vi "IMAQdx_AbsImage_Flea3_v4.3.vi"() -> ()   [LabVIEW 2012]
doc: "Take a single PixelFly exposure and display the result as an intensity graph.This VI illustrates the basics of taking an exposure with the PixelFly camera. Use Ctrl-H to get help on any of the controls\n\nCopyright 2001, The Cooke Corporation."
uses:
  LabVIEW Data V4.10/Shared Libraries/Controls/FileName_Cluster.ctl
  <vilib>/userdefined/High Color/IMAQdx.ctl
  <vilib>/vision/driver/IMAQdx.llb/IMAQdx Acquisition Mode.ctl
  Shared Libraries/Controls/FileInfo_Global.vi
  <vilib>/Analysis/NI_AALBase.lvlib
  <vilib>/vision/driver/NI_Vision_Acquisition_Software.lvlib
panel:
  in  "Interrupt":bool
  out "Buffer Number":u32=4294967294
  out "Frames":i32
  out "Loop":i32=292
  out "Status":string="Running..."
  in  "stop":bool
  in  "Tab Control":enum32{"Setup", "Images", "Hardware status"}(tab)=enum."Images"
  in  "Camera Name":T1="Flr XZ"
  in  "Experiment":T2(ring)=enum."Sr"
  in  "Accept parameters from remote system":bool=TRUE
  in  "Bias (Amps)":dbl
  in  "Pinch Coil (Amps)":dbl=520.0
  in  "Expansion time (ms)":dbl=19.0
  in  "Trap min at 0 (MHz)":dbl=2.85
  in  "Detuning (Linewidths)":dbl
  in  "Racetrack (Amps)":dbl=540.0
  in  "Magnification":dbl=0.399
  in  "Image direction":enum16{"XY", "XZ"}(ring)=enum."XZ"
  in  "Imaging technique":enum16{"Absorption", "Fluorescence", "RawImage"}(ring)
  in  "File Parameters":T3={"Data Root"=path "C:/Experiment/Data", "Index"=20503, "Instrument"="Flea3_20S4M"} {"Index" format="%04d"}
  in  "Send data to Igor?":bool=TRUE
  out "Command to Igor":string="AutoRunV3(\"rMOTDet_Sr_88\",\"C:\\\\Experiment\\\\Data\\\\2013\\\\October\\\\09\\\\Flea3_20S4M_09Oct2013_20502.ibw\") "
  out "Image note":string="Experiment=Sr\nCamera_ID=Flea3_20S4M\nImageType=Raw\nDataType=Absorption\nImageDirection=XZ\nMagnification=3.990000E-1\nFileNumber=20502\n# Current Variables\n# \nplus_zman=-1.971000E+0\nminus_zman=-1.584000E+0\ncompensation=-8.000000E-1\nXshim=4.000000E-1\nYshim=1.200000E+0\nZshim=9.000000E-1\nProbePow=1.600000E+0\ntau=0.000000E+0\ntEnd=0.000000E+0\nDipStart=0.000000E+0\nMOTcurrent=-1.500000E+0\nProbeDet=0.000000E+0\nTOF=1.000000E-4\nMOTPow=8.000000E+0\nMOTdetuning=-4.500000E+1\nRampTau=2.000000E-3\nPf=1.900000E+0\nrMOTcurr=-7.500000E-2\nrMOTcurrI=-5.000000E-2\nrMOTcurrF=-5.000000E-2\ncombWidthI=4.000000E+0\ncombWidthF=5.000000E-1\nrMOTbroadDetuning=2.750000E+0\nrMOTsat1=1.500000E+4\nrMOTsat2=1.000000E+3\nrMOTsat3=1.500000E+2\nsingleFreqDet=1.000000E+3\nPdet=3.500000E+0\nZshimVar=9.000000E-1\n# Master Staging List\n# Line\tMarker\tOption\tHalt\t0       4       8      12      16      20    AO\tDelay\t\tPoints\t0\t\t1\t\t2\t\t3\t\t4\t\t5\t\t6\t\t7\t\t8\t\t9\t\t10\t\t11\t\t12\t\t13\t\t14\t\t15\t\tComment\n00\t\tRamp\t1 0 0 0 0 0 1 0 0 0 1 1 1 1 1 0 0 0 0 0 0 0 0 0\t.1\t0\tplus_zman\tminus_zman\tcompensation\tMOTcurrent\trMOTsat(rMOTsat1)\tcombAmplitude(combWidthI)\trMOTdelta(-(rMOTbroadDetuning +combWidthI/2))\t2.65\tbMOTdelta(MOTdetuning)\tbMOTpow(0.5)\tProbePow\tPdelta(Pdet)\tXshim\tYshim\tZshim\t0\treset\n01\t\tRamp\t1 1 0 0 0 0 0 0 0 0 1 1 1 1 1 1 0 0 0 0 0 0 0 0\t3\t0\tplus_zman\tminus_zman\tcompensation\tMOTcurrent\trMOTsat(rMOTsat1)\tcombAmplitude(combWidthI)\trMOTdelta(-(rMOTbroadDetuning +combWidthI/2))\t2.65\tbMOTdelta(MOTdetuning)\tbMOTpow(MOTPow)\tProbePow\tPdelta(Pdet)\tXshim\tYshim\tZshim\t0\tblue MOT load\n02\t\tRamp\t1 1 0 0 0 0 0 0 0 0 1 1 1 1 1 1 0 0 0 0 0 0 0 0\t0.000244\t0\tplus_zman\tminus_zman\tcompensation\tMOTcurrent\trMOTsat(rMOTsat1)\tcombAmplitude(combWidthI)\trMOTdelta(-(rMOTbroadDetuning +combWidthI/2))\t2.65\tbMOTdelta(MOTdetuning)\tbMOTpow(MOTPow)\tProbePow\tPdelta(Pdet)\tXshim\tYshim\tZshim\t0\tpretrig\n03\t\tRamp\t1 1 0 0 0 0 0 0 0 0 1 1 1 1 1 1 0 0 0 0 0 0 0 0\t0.074\t0\tplus_zman\tminus_zman\tcompensation\tMOTcurrent\trMOTsat(rMOTsat1)\tcombAmplitude(combWidthI)\trMOTdelta(-(rMOTbroadDetuning +combWidthI/2))\t2.65\tbMOTdelta(MOTdetuning)\tbMOTpow(MOTPow)\tProbePow\tPdelta(Pdet)\tXshim\tYshim\tZshim\t0\tCamWaitTime\n04\t\tRamp\t1 1 0 0 0 0 0 0 0 0 1 1 1 1 1 1 0 0 0 0 0 0 0 0\t0.001120\t0\tplus_zman\tminus_zman\tcompensation\tMOTcurrent\trMOTsat(rMOTsat1)\tcombAmplitude(combWidthI)\trMOTdelta(-(rMOTbroadDetuning +combWidthI/2))\t2.65\tbMOTdelta(MOTdetuning)\tbMOTpow(MOTPow)\tProbePow\tPdelta(Pdet)\tXshim\tYshim\tZshim\t0\tProbeShutOn\n05\t\tRamp\t1 1 0 0 0 0 0 0 0 0 1 1 1 1 1 1 0 0 0 0 0 0 0 0\t0.000260\t0\tplus_zman\tminus_zman\tcompensation\tMOTcurrent\trMOTsat(rMOTsat1)\tcombAmplitude(combWidthI)\trMOTdelta(-(rMOTbroadDetuning +combWidthI/2))\t2.65\tbMOTdelta(MOTdetuning)\tbMOTpow(MOTPow)\tProbePow\tPdelta(Pdet)\tXshim\tYshim\tZshim\t0\tRepumpShutOff\n06\t\tRamp\t1 1 0 0 0 0 1 0 0 0 1 1 1 1 1 1 0 0 0 0 0 0 0 0\t0.001370\t0\tplus_zman\tminus_zman\tcompensation\tMOTcurrent\trMOTsat(rMOTsat1)\tcombAmplitude(combWidthI)\trMOTdelta(-(rMOTbroadDetuning +combWidthI/2))\t2.65\tbMOTdelta(MOTdetuning)\tbMOTpow(MOTPow)\tProbePow\tPdelta(Pdet)\tXshim\tYshim\tZshim\t0\tMOTShutOff\n07\t\tRamp\t1 1 0 0 0 0 1 0 0 0 1 1 1 1 0 0 0 0 0 0 0 0 0 0\t0.000230\t0\tplus_zman\tminus_zman\tcompensation\trMOTcurrI\trMOTsat(rMOTsat1)\tcombAmplitude(combWidthI)\trMOTdelta(-(rMOTbroadDetuning +combWidthI/2))\t2.65\tbMOTdelta(MOTdetuning)\tbMOTpow(0.5)\tProbePow\tPdelta(Pdet)\tXshim\tYshim\tZshim\t0\tCoil Switch\n08\t\tRamp\t1 1 0 0 0 0 1 0 0 0 1 1 0 0 0 0 0 0 0 0 0 0 0 0\t.1\t0\tplus_zman\tminus_zman\tcompensation\trMOTcurrI\trMOTsat(rMOTsat1)\tcombAmplitude(combWidthI)\trMOTdelta(-(rMOTbroadDetuning +combWidthI/2))\t2.65\tbMOTdelta(MOTdetuning)\tbMOTpow(0.5)\tProbePow\tPdelta(Pdet)\tXshim\tYshim\tZshim\t0\tCapture Red MOT\n09\t\tRamp\t1 1 0 0 0 0 1 0 0 0 1 1 0 0 0 0 0 0 0 0 0 0 0 0\t.1\t0\tplus_zman\tminus_zman\tcompensation\trMOTcurrI\tLineRamp(f,rMOTsat(rMOTsat1),rMOTsat(rMOTsat2))\tLineRamp(f,combAmplitude(combWidthI),combAmplitude(combWidthF))\tLineRamp(f,rMOTdelta(-(rMOTbroadDetuning +combWidthI/2)),rMOTdelta(-(rMOTbroadDetuning +combWidthF/2)))\t2.65\tbMOTdelta(MOTdetuning)\tbMOTpow(0.5)\tProbePow\tPdelta(Pdet)\tXshim\tYshim\tZshim\t0\tRamp broad rMOT\n10\t\tRamp\t1 1 0 0 0 0 1 0 0 0 1 1 0 0 0 0 0 0 0 0 0 0 0 0\t.05\t0\tplus_zman\tminus_zman\tcompensation\trMOTcurrI\trMOTsat(rMOTsat2)\tcombAmplitude(combWidthF)\trMOTdelta(-(rMOTbroadDetuning +combWidthF/2))\t2.65\tbMOTdelta(MOTdetuning)\tbMOTpow(0.5)\tProbePow\tPdelta(Pdet)\tXshim\tYshim\tLineRamp(f,Zshim,ZshimVar)\t0\tRamp broad rMOT\n11\t\tRamp\t1 1 0 0 0 0 1 0 0 0 1 1 0 0 0 0 0 0 0 0 0 0 0 0\t.1\t0\tplus_zman\tminus_zman\tcompensation\trMOTcurrI\trMOTsat(rMOTsat2)\tcombAmplitude(combWidthF)\trMOTdelta(-(rMOTbroadDetuning +combWidthF/2))\t2.65\tbMOTdelta(MOTdetuning)\tbMOTpow(0.5)\tProbePow\tPdelta(Pdet)\tXshim\tYshim\tZshimVar\t0\tRamp broad rMOT\n12\t\tRamp\t1 1 0 0 0 0 1 1 1 1 0 1 0 0 0 0 0 0 0 0 0 0 0 0\tTOF\t0\tplus_zman\tminus_zman\tcompensation\trMOTcurrF\trMOTsat(rMOTsat3)\tcombAmplitude(combWidthF)\trMOTdelta(-(rMOTbroadDetuning +combWidthF/2))\t2.65\tbMOTdelta(MOTdetuning)\tbMOTpow(0.5)\tProbePow\tPdelta(Pdet)\tXshim\tYshim\tZshimVar\t0\tTOF\n13\t\tRamp\t1 1 0 0 0 0 1 1 1 1 0 1 0 0 0 0 0 0 0 0 0 0 0 0\t.000044\t0\tplus_zman\tminus_zman\tcompensation\trMOTcurrF\trMOTsat(rMOTsat3)\tcombAmplitude(combWidthI)\trMOTdelta(-(rMOTbroadDetuning +combWidthI/2))\t2.65\tbMOTdelta(MOTdetuning)\tbMOTpow(0.5)\tProbePow\tPdelta(Pdet)\tXshim\tYshim\tZshimVar\t0\tarm camera\n14\t\tRamp\t1 1 0 0 0 0 1 1 1 1 0 1 0 1 0 0 0 0 0 0 0 0 0 0\t.000200\t0\tplus_zman\tminus_zman\tcompensation\trMOTcurrF\trMOTsat(rMOTsat3)\tcombAmplitude(combWidthI)\trMOTdelta(-(rMOTbroadDetuning +combWidthI/2))\t2.65\tbMOTdelta(MOTdetuning)\tbMOTpow(0.5)\tProbePow\tPdelta(Pdet)\tXshim\tYshim\tZshimVar\t0\tatom img\n15\t\tRamp\t1 0 0 0 0 0 1 1 1 1 1 1 0 0 0 0 0 0 0 0 0 0 0 0\t.07\t0\tplus_zman\tminus_zman\tcompensation\trMOTcurrF\trMOTsat(rMOTsat3)\tcombAmplitude(combWidthI)\trMOTdelta(-(rMOTbroadDetuning +combWidthI/2))\t2.65\tbMOTdelta(MOTdetuning)\tbMOTpow(0.5)\tProbePow\tPdelta(Pdet)\tXshim\tYshim\tZshimVar\t0\ttransmit img\n16\t\tRamp\t0 0 0 0 0 0 1 1 1 1 1 1 0 0 1 1 0 0 0 0 0 0 0 0\t.000044\t0\tplus_zman\tminus_zman\tcompensation\trMOTcurrF\trMOTsat(rMOTsat3)\tcombAmplitude(combWidthI)\trMOTdelta(-(rMOTbroadDetuning +combWidthI/2))\t2.65\tbMOTdelta(MOTdetuning)\tbMOTpow(0.5)\tProbePow\tPdelta(Pdet)\tXshim\tYshim\tZshimVar\t0\tarm camera\n17\t\tRamp\t0 0 0 0 0 0 1 1 1 1 1 1 0 1 1 1 0 0 0 0 0 0 0 0\t.000200\t0\tplus_zman\tminus_zman\tcompensation\trMOTcurrF\trMOTsat(rMOTsat1)\tcombAmplitude(combWidthI)\trMOTdelta(-(rMOTbroadDetuning +combWidthI/2))\t2.65\tbMOTdelta(MOTdetuning)\tbMOTpow(0.5)\tProbePow\tPdelta(Pdet)\tXshim\tYshim\tZshimVar\t0\tprobe img\n18\t\tRamp\t0 0 0 0 0 0 1 1 1 1 1 1 0 0 1 1 0 0 0 0 0 0 0 0\t.07\t0\tplus_zman\tminus_zman\tcompensation\trMOTcurrF\trMOTsat(rMOTsat1)\tcombAmplitude(combWidthI)\trMOTdelta(-(rMOTbroadDetuning +combWidthI/2))\t2.65\tbMOTdelta(MOTdetuning)\tbMOTpow(0.5)\tProbePow\tPdelta(Pdet)\tXshim\tYshim\tZshimVar\t0\ttransmit img\n19\t\tRamp\t0 0 0 0 0 0 1 1 1 1 1 1 0 0 1 1 0 0 0 0 0 0 0 0\t.000044\t0\tplus_zman\tminus_zman\tcompensation\trMOTcurrF\trMOTsat(rMOTsat1)\tcombAmplitude(combWidthI)\trMOTdelta(-(rMOTbroadDetuning +combWidthI/2))\t2.65\tbMOTdelta(MOTdetuning)\tbMOTpow(0.5)\tProbePow\tPdelta(Pdet)\tXshim\tYshim\tZshimVar\t0\tarm camera\n20\t\tRamp\t0 0 0 0 0 0 1 1 1 1 1 1 0 0 1 1 0 0 0 0 0 0 0 0\t.000200\t0\tplus_zman\tminus_zman\tcompensation\trMOTcurrF\trMOTsat(rMOTsat1)\tcombAmplitude(combWidthI)\trMOTdelta(-(rMOTbroadDetuning +combWidthI/2))\t2.65\tbMOTdelta(MOTdetuning)\tbMOTpow(0.5)\tProbePow\tPdelta(Pdet)\tXshim\tYshim\tZshimVar\t0\tbg img\n21\t\tRamp\t0 0 0 0 0 0 1 1 1 1 1 1 0 0 1 1 0 0 0 0 0 0 0 0\t.07\t0\tplus_zman\tminus_zman\tcompensation\tMOTcurrent\trMOTsat(rMOTsat1)\tcombAmplitude(combWidthI)\trMOTdelta(-(rMOTbroadDetuning +combWidthI/2))\t2.65\tbMOTdelta(MOTdetuning)\tbMOTpow(0.5)\tProbePow\tPdelta(Pdet)\tXshim\tYshim\tZshimVar\t0\ttransmit img\n22\t\tRamp\t0 0 0 0 0 0 1 0 0 0 1 1 1 1 1 1 0 0 0 0 0 0 0 0\t0.5\t0\tplus_zman\tminus_zman\tcompensation\tMOTcurrent\trMOTsat(rMOTsat1)\tcombAmplitude(combWidthI)\trMOTdelta(-(rMOTbroadDetuning +combWidthI/2))\t2.65\tbMOTdelta(MOTdetuning)\tbMOTpow(MOTPow)\tProbePow\tPdelta(Pdet)\tXshim\tYshim\tZshimVar\t0\talignment\n# Slave Staging List\n# Line\tMarker\tOption\tHalt\t0       4       8      12      16      20    AO\tDelay\t\tPoints\t0\t\t1\t\t2\t\t3\t\t4\t\t5\t\t6\t\t7\t\t8\t\t9\t\t10\t\t11\t\t12\t\t13\t\t14\t\t15\t\tComment\n# SRS List\n# \n#\n# Evaporation\n\nDDS Table\r\n"
  in  "Igor Wave Name":string="Test_Img"
  in  "Save file to archive?":bool=TRUE
  in  "Timeout (ms)":u32=10000
  in  "Gain":dbl
  in  "Shutter speed":dbl=0.03
  out "Timeout":bool=TRUE
  out "Trigger Overrun":bool=TRUE
  in  "Quad [Amps]":dbl=540.0
  in  "Source of File Data":refnum<k21>="\\\\Control\\VariableLibrary\\Instruction String"
  in  "Bits to shift":i32
  in  "Raw image to view":u16(ring)=1 items=["Clear", "Absorbtion", "Probe", "Background"]
  in  "Update Graphics":bool=TRUE
  out "Raw Image":u16[][](graph)
  out "Processed Image":sgl[][](graph)
  out "Histogram":cluster{"X Values":dbl[], dbl[]}(graph)={"X Values"=[33.3203125, 83.9609375, 134.6015625, 185.2421875, 235.8828125, 286.5234375, 337.1640625, 387.8046875, 438.4453125, 489.0859375, 539.7265625, 590.3671875, 641.0078125, 691.6484375, 742.2890625, 792.9296875, 843.5703125, 894.2109375, 944.8515625, 995.4921875, 1046.1328125, 1096.7734375, 1147.4140625, 1198.0546875, 1248.6953125, 1299.3359375, 1349.9765625, 1400.6171875, 1451.2578125, 1501.8984375, 1552.5390625, 1603.1796875, 1653.8203125, 1704.4609375, 1755.1015625, 1805.7421875, 1856.3828125, 1907.0234375, 1957.6640625, 2008.3046875, 2058.9453125, 2109.5859375, 2160.2265625, 2210.8671875, 2261.5078125, 2312.1484375, 2362.7890625, 2413.4296875, 2464.0703125, 2514.7109375, 2565.3515625, 2615.9921875, 2666.6328125, 2717.2734375, 2767.9140625, 2818.5546875, 2869.1953125, 2919.8359375, 2970.4765625, 3021.1171875, 3071.7578125, 3122.3984375, 3173.0390625, 3223.6796875], [3.7989267385772014, 4.5429374082326195, 4.748110467494984, 4.839886381275089, 4.874528201815916, 4.882473307537075, 4.900061102735481, 4.901899475590769, 4.901322072145771, 4.91365493508662, 4.918664530902084, 4.913633741719355, 4.9192611900011745, 4.903768042526874, 4.9022368466531665, 4.881578647766411, 4.85617283090403, 4.839697967180202, 4.816519689651045, 4.788479480483438, 4.776606761880874, 4.7497285878404885, 4.705264862317404, 4.681819910988056, 4.644999560017717, 4.606370615114146, 4.576064788225377, 4.5289423974157295, 4.494182432516058, 4.452629651622018, 4.390139938467622, 4.355432362470549, 4.299746933493803, 4.233478391931892, 4.179666668690498, 4.114377429786155, 4.018325945402921, 3.9655309436228605, 3.874423830586502, 3.8100307864058394, 3.713994267660644, 3.6097011023793995, 3.5090680450171616, 3.3694014136966244, 3.248218561190075, 3.118264726089479, 2.9836262871245345, 2.8228216453031045, 2.6748611407378116, 2.53655844257153, 2.342422680822206, 2.173186268412274, 2.0253058652647704, 1.7993405494535817, 1.5797835966168101, 1.146128035678238, 1.2304489213782739, 0.6020599913279624, 0.8450980400142568, 0.8450980400142568, 0.9030899869919435, 0.8450980400142568, 0.0, 0.47712125471966244]}
  out "Images":u16[][][](array[numeric])
  out "Camera Error":errorcluster={"status"=FALSE, "code"=-1074360293, "source"="IMAQdx Get Image.vi"}
  out "DDE Error":errorcluster={"status"=FALSE, "code"=0, "source"="DDE Close: No Error"}
  out "Status Array":T4(array[cluster])=[{"AcquisitionInProgress"=FALSE, "BufferCount"=4, "LastBufferNumber"=3, "LostBufferCount"=0}, {"AcquisitionInProgress"=TRUE, "BufferCount"=1, "LastBufferNumber"=0, "LostBufferCount"=0}, {"AcquisitionInProgress"=TRUE, "BufferCount"=2, "LastBufferNumber"=1, "LostBufferCount"=0}, {"AcquisitionInProgress"=TRUE, "BufferCount"=3, "LastBufferNumber"=2, "LostBufferCount"=0}, {"AcquisitionInProgress"=TRUE, "BufferCount"=4, "LastBufferNumber"=3, "LostBufferCount"=0}]
  # "Flea3 Image Acquisition v4.3"
  # "Experimental Paramaters"
  # "Cam0 is XZ, Cam1 is XY"
  # "RbYb: set to 0."
  # "The only get set on 1st run.\nUse  a Gain of 10:\n* Seems to give a readout error of 1 bit.\n* Know intensity calibration"
  # "In both techniques 3 images\nare aquired, but in Fluorescense\nthe 3rd is discarded"
  # "Sr: .663  is XZ\n     5.48 is XY"
  # "Obsolete: (now done with network variables)\nWhen paramaters are accepted from a remote system a DataSockets server\nmust be running on this machine (in start menu in National Instruments folder)"
  # "Camera configuration"
  # "File configuration"
  # "When the gain is 10 :  742 counts = Isat with 100 us pulse.  This is fine and\nis the point of highest SNR.  Linearized in software."
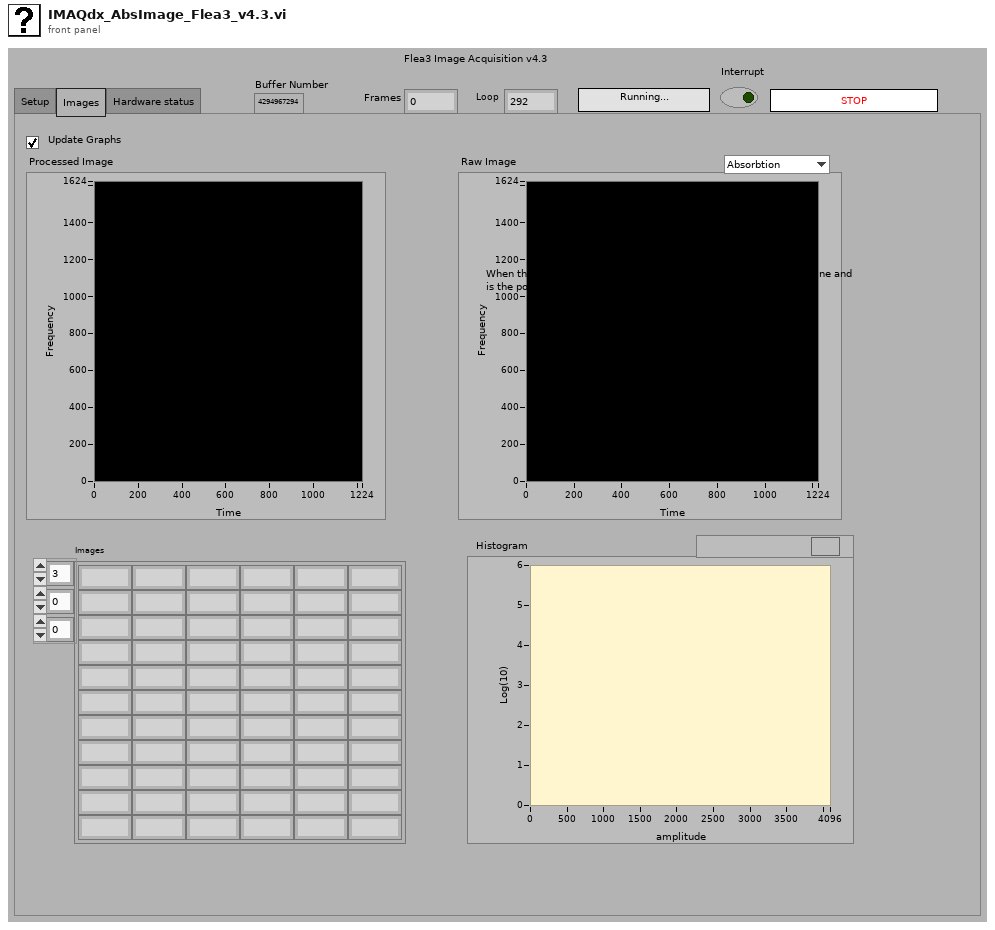
[diagram p1: front panel]
types:
  T1 = typedef "IMAQdx.ctl" = refnum<k21>
  T2 = enum16{"Rubidium I", "Rubidium II", "RbLi", "RbYb", "Sr"}
  T3 = typedef "FileName_Cluster.ctl" = cluster{"Data Root":path, "Index":u32, "Instrument":string}
  T4 = cluster{"AcquisitionInProgress":bool, "BufferCount":u32, "LastBufferNumber":u32, "LostBufferCount":u32}[]
  T5 = typedef "NI_Vision_Acquisition_Software.lvlib/IMAQdx Acquisition Mode.ctl" = enum32{"One Shot", "Continuous"}
  T6 = typedef "Image Type" = u32
  T7 = typedef "IMAQ Image.ctl" = refnum<image>
  T8 = cluster{"AcquisitionInProgress":bool, "BufferCount":u32, "LastBufferNumber":u32, "LostBufferCount":u32}
  T9 = cluster{"X Values":dbl[], "Histogram: h(x)":i32[]}
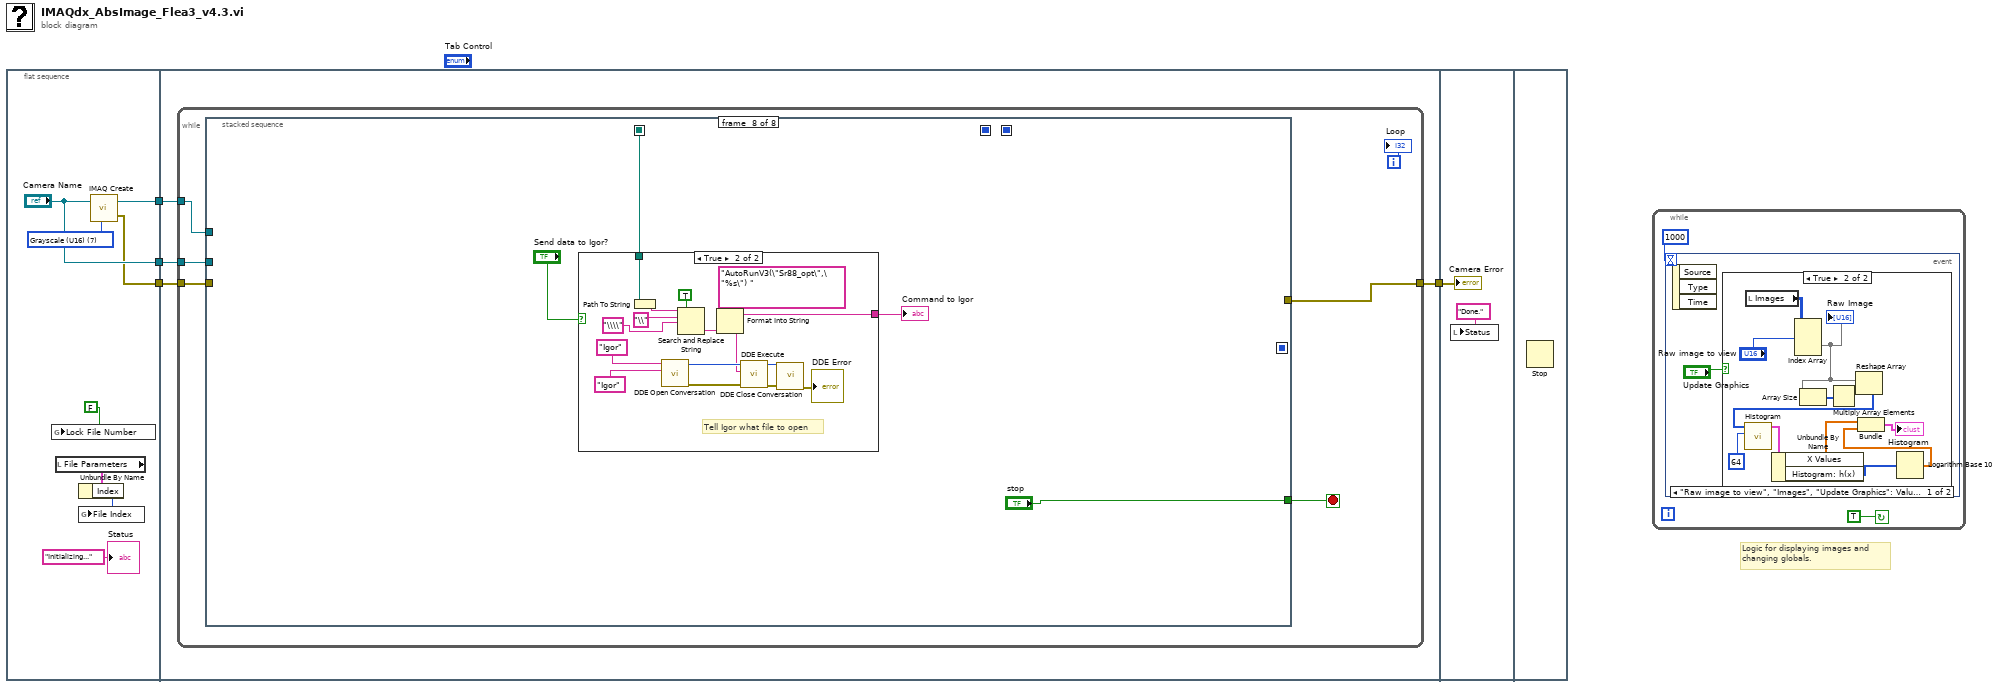
[diagram p0: block diagram]
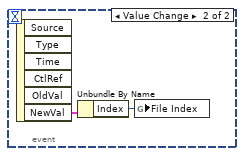
[diagram p3: hidden frame]
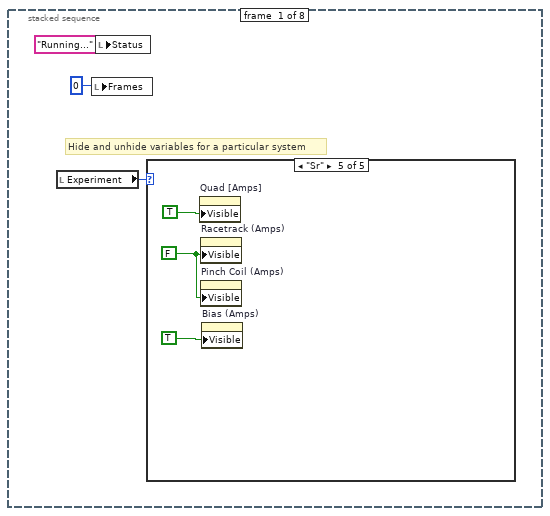
[diagram p4: hidden frame]
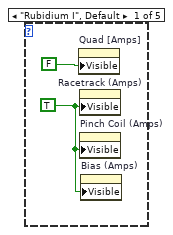
[diagram p5: hidden frame]
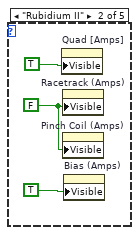
[diagram p6: hidden frame]
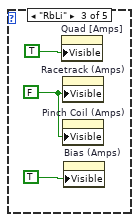
[diagram p7: hidden frame]
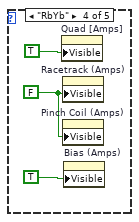
[diagram p8: hidden frame]
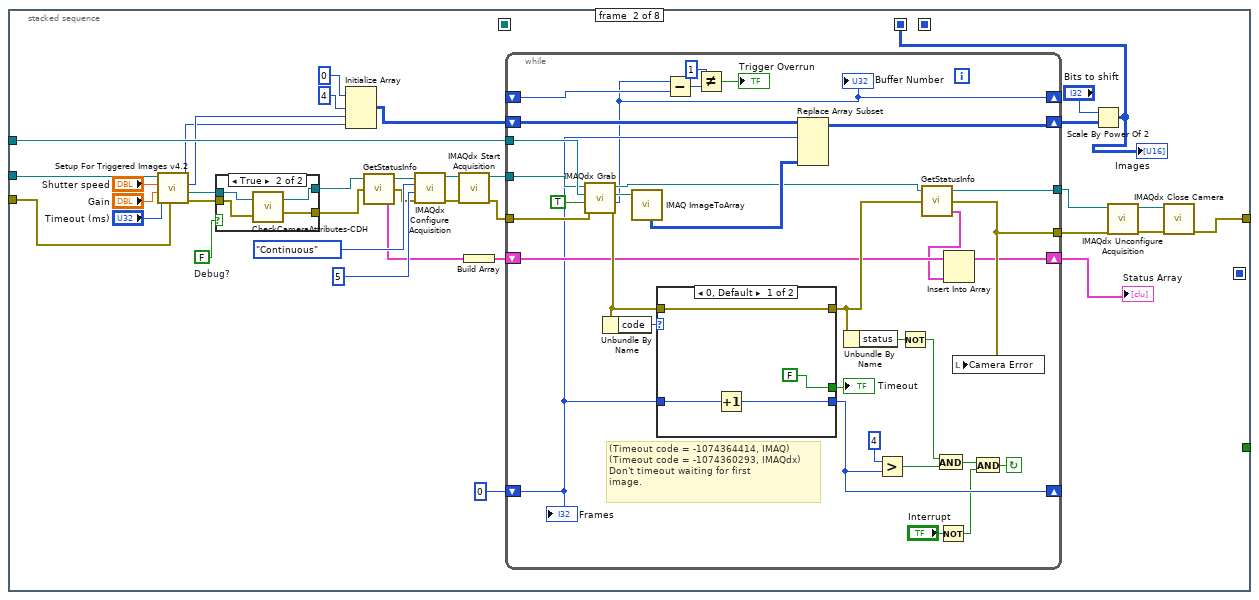
[diagram p9: hidden frame]
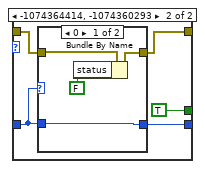
[diagram p11: hidden frame]
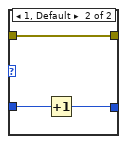
[diagram p12: hidden frame]
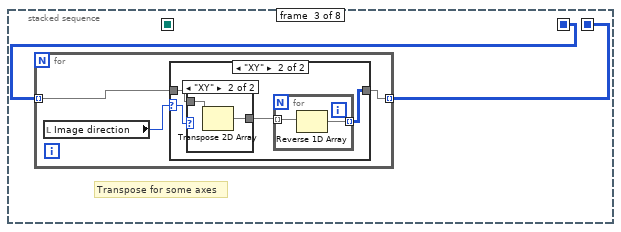
[diagram p13: hidden frame]
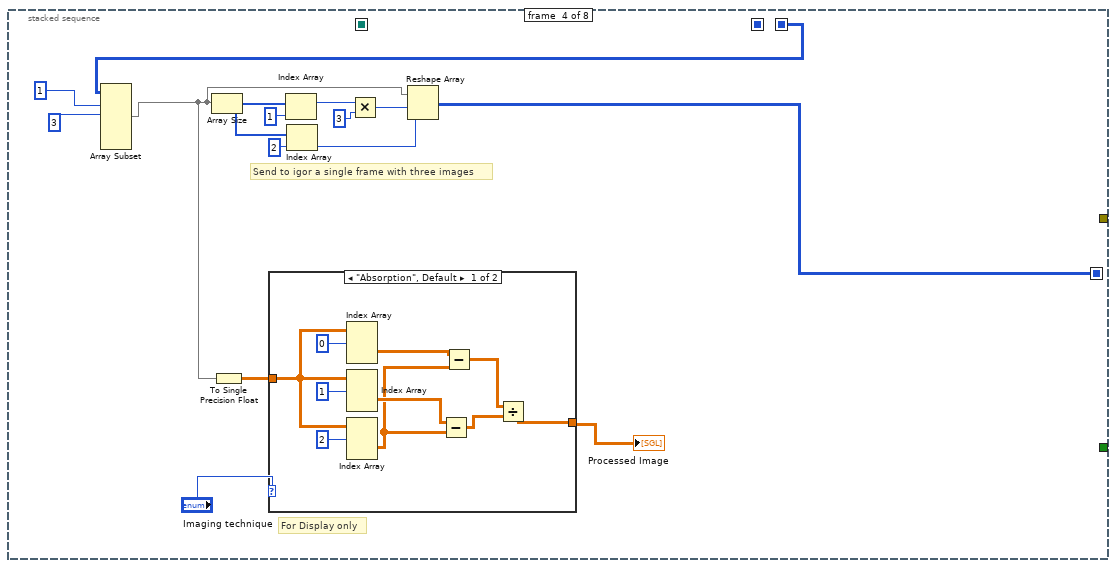
[diagram p16: hidden frame]
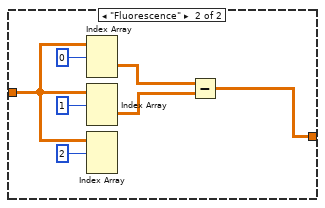
[diagram p17: hidden frame]
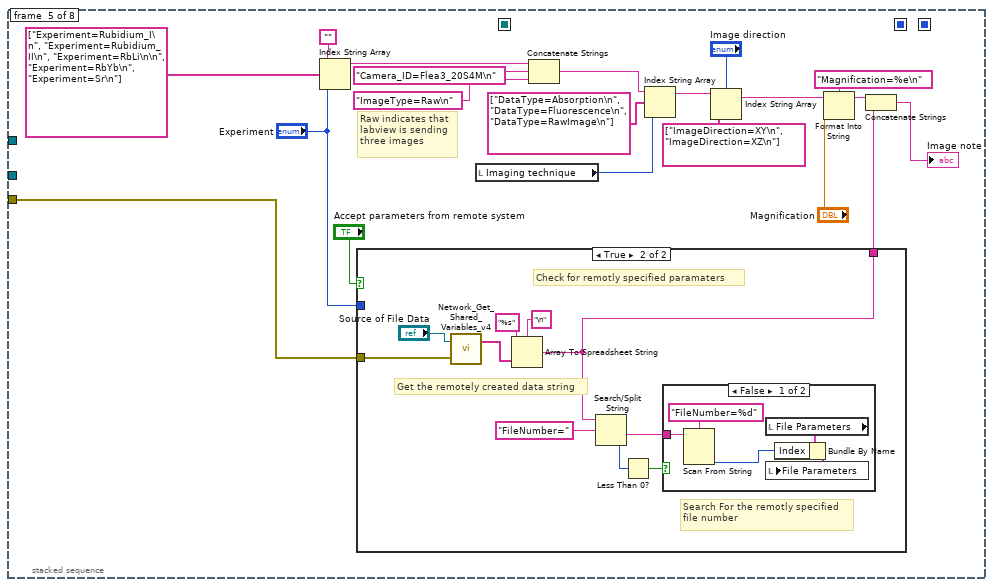
[diagram p18: hidden frame]
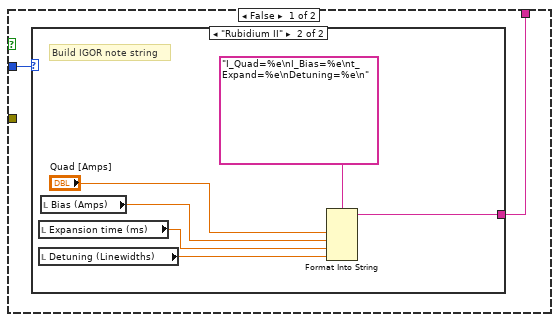
[diagram p19: hidden frame]
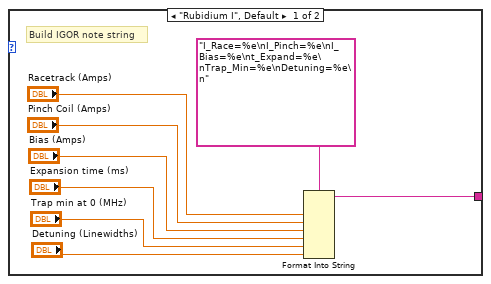
[diagram p20: hidden frame]
diagram:
  # "Logic for displaying images and\nchanging globals."
  n1 = flat-sequence {
    tunnel: [w8] -> w4
    tunnel: ["Camera Name"] -> w3
    tunnel: [w6] -> w2
    tunnel: w3 -> [w16]
    tunnel: w4 -> [w15]
    tunnel: w2 -> [w14]
    tunnel: [w13] -> w1
    tunnel: w1 -> [w261]
    frame #0 {
      w5 = T6 7 items=["Grayscale (U8)", "Grayscale (I16)", "Grayscale (SGL)", "Complex (CSG)", "RGB (U32)", "HSL (U32)", "RGB (U64)", "Grayscale (U16)"] ("Image Type")
      n2 = global write "FileInfo_Global.vi" "Lock File Number"(FALSE) -> ()
      n3 = local read "File Parameters"() -> (w9:T3)
      n4 = Unbundle By Name(w9) -> ("Index"=w10:u32)
      n5 = global write "FileInfo_Global.vi" "File Index"(w10) -> ()
      n6 = call "IMAQ Create"("Image Name"="Camera Name", "Image Type"=w5) -> ("New Image"=w8:T7, "error out"=w6:errorcluster)  [unwired: 2 in, 1 out]
      "Status" <- "Initializing..."
    }
    frame #1 {
      n7 = while {
        tunnel: w16 -> [w19]
        tunnel: w15 -> [w20]
        tunnel: w14 -> [w18]
        tunnel: [w17] -> w13
        i -> [w22]
        stop <- w21 stop-if-true
        n8 = stacked-sequence {
          seq-local: [_ _ _ w158 _ _ _ _] -> [_ _ _ _ _ w233 _ _]
          seq-local: [_ _ _ _ _ w229 _ _] -> [_ _ _ _ _ _ _ w243]
          seq-local: [_ w60 _ _ _ _ _ _] -> [_ _ w132 _ _ _ _ _]
          seq-local: [_ _ w131 _ _ _ _ _] -> [_ _ _ w149 _ _ _ _]
          tunnel: [_ _ _ _ _ _ _ "stop"] -> w21
          tunnel: w18 -> [_ w66 _ _ w185 _ _ _]
          tunnel: w19 -> [_ w67 _ _ _ _ _ _]
          tunnel: w20 -> [_ w75 _ _ _ _ _ _]
          tunnel: [_ w65 _ _ _ _ _ _] -> w17
          frame #0 {
            # "Hide and unhide variables for a particular system"
            n9 = local read "Experiment"() -> (w23:T2)
            n10 = local write "Frames"(0) -> ()
            n11 = local write "Status"("Running...") -> ()
            n12 = case shown="\"Sr\"" w23 {
              frame "Rubidium I", Default {
                w26 = TRUE
                n13 = property on="Quad [Amps]" class="DigNum (strict)"("Visible"=FALSE) -> ()  [unwired: 2 in, 2 out]
                n14 = property on="Racetrack (Amps)" class="DigNum (strict)"("Visible"=w26) -> ()  [unwired: 2 in, 2 out]
                n15 = property on="Pinch Coil (Amps)" class="DigNum (strict)"("Visible"=w26) -> ()  [unwired: 2 in, 2 out]
                n16 = property on="Bias (Amps)" class="DigNum (strict)"("Visible"=w26) -> ()  [unwired: 2 in, 2 out]
              }
              frame "Rubidium II" {
                w29 = FALSE
                n17 = property on="Quad [Amps]" class="DigNum (strict)"("Visible"=TRUE) -> ()  [unwired: 2 in, 2 out]
                n18 = property on="Racetrack (Amps)" class="DigNum (strict)"("Visible"=w29) -> ()  [unwired: 2 in, 2 out]
                n19 = property on="Pinch Coil (Amps)" class="DigNum (strict)"("Visible"=w29) -> ()  [unwired: 2 in, 2 out]
                n20 = property on="Bias (Amps)" class="DigNum (strict)"("Visible"=TRUE) -> ()  [unwired: 2 in, 2 out]
              }
              frame "RbLi" {
                w32 = FALSE
                n21 = property on="Quad [Amps]" class="DigNum (strict)"("Visible"=TRUE) -> ()  [unwired: 2 in, 2 out]
                n22 = property on="Racetrack (Amps)" class="DigNum (strict)"("Visible"=w32) -> ()  [unwired: 2 in, 2 out]
                n23 = property on="Pinch Coil (Amps)" class="DigNum (strict)"("Visible"=w32) -> ()  [unwired: 2 in, 2 out]
                n24 = property on="Bias (Amps)" class="DigNum (strict)"("Visible"=TRUE) -> ()  [unwired: 2 in, 2 out]
              }
              frame "RbYb" {
                w35 = FALSE
                n25 = property on="Quad [Amps]" class="DigNum (strict)"("Visible"=TRUE) -> ()  [unwired: 2 in, 2 out]
                n26 = property on="Racetrack (Amps)" class="DigNum (strict)"("Visible"=w35) -> ()  [unwired: 2 in, 2 out]
                n27 = property on="Pinch Coil (Amps)" class="DigNum (strict)"("Visible"=w35) -> ()  [unwired: 2 in, 2 out]
                n28 = property on="Bias (Amps)" class="DigNum (strict)"("Visible"=TRUE) -> ()  [unwired: 2 in, 2 out]
              }
              frame "Sr" {
                w38 = FALSE
                n29 = property on="Quad [Amps]" class="DigNum (strict)"("Visible"=TRUE) -> ()  [unwired: 2 in, 2 out]
                n30 = property on="Racetrack (Amps)" class="DigNum (strict)"("Visible"=w38) -> ()  [unwired: 2 in, 2 out]
                n31 = property on="Pinch Coil (Amps)" class="DigNum (strict)"("Visible"=w38) -> ()  [unwired: 2 in, 2 out]
                n32 = property on="Bias (Amps)" class="DigNum (strict)"("Visible"=TRUE) -> ()  [unwired: 2 in, 2 out]
              }
            }
          }
          frame #1 {
            w53 = FALSE  # Debug?
            n33 = call "Setup For Triggered Images v4.2.vi"("error in"=w66, "Timeout (ms)"="Timeout (ms)", "Gain"="Gain", "Shutter speed"="Shutter speed", "Camera Name"=w67) -> ("Error out"=w54:errorcluster, "Session Out"=w55:T1, "Height"=w64:u32, "Width"=w63:u32)
            n34 = case shown="True" w53 {
              tunnel: [w76 w81] -> w49
              tunnel: [w77 w80] -> w46
              tunnel: w55 -> [w76 w79]
              tunnel: w54 -> [w77 w78]
              frame False {
              }
              frame True {
                n35 = call "CheckCameraAttributes-CDH.vi"("error in"=w78, "Camera Name"=w79) -> ("error out"=w80:errorcluster, "Session Out"=w81:T1)
              }
            }
            n36 = Initialize Array(u16 0, 4, w64, w63) -> (w71:u16[][][])
            n37 = call "GetStatusInfo.vi"("error in"=w46, "Camera In"=w49) -> ("Status Info"=w45:T8, "error out"=w47:errorcluster, "Camera Out"=w48:T1)  [unwired: 1 in]
            n38 = call <vilib>:"IMAQdx Configure Acquisition.vi"("error in"=w47, "Number of Buffers"=u32 5, "Continuous?"=IMAQdx_Acquisition_Mode."Continuous", "Session In"=w48) -> ("error out"=w56:errorcluster, "Session Out"=w57:T1)  [unwired: 6 in]
            n39 = call <vilib>:"IMAQdx Start Acquisition.vi"("error in"=w56, "Session In"=w57) -> ("error out"=w50:errorcluster, "Session Out"=w51:T1)  [unwired: 8 out]
            n40 = Build Array(w45) -> (w52:T4)
            n41 = while {
              tunnel: w75 -> [w104]
              shift-right: [w82] -> _
              shift-left: _ -> [w109]
              tunnel: [w90] -> w43
              tunnel: w50 -> [w102]
              tunnel: [w87] -> w41
              shift-right: [w97] -> _
              shift-left: 0 -> [w84]
              shift-right: [w105] -> w61
              shift-left: w71 -> [w106]
              tunnel: w51 -> [w103]
              shift-right: [w85] -> w44
              shift-left: w52 -> [w86]
              stop <- w93 continue-if-true
              # "(Timeout code = -1074364414, IMAQ)\n(Timeout code = -1074360293, IMAQdx)\nDon't timeout waiting for first\nimage."
              n42 = call <vilib>:"IMAQdx Grab.vi"("error in"=w102, "Wait for Next Buffer? (Yes)"=TRUE, "Image In"=w104, "Session In"=w103) -> ("error out"=w101:errorcluster, "Buffer Number Out"=w82:u32, "Image Out"=w96:T7, "Session Out"=w89:T1)  [unwired: 4 out]
              "Buffer Number" <- w82
              n43 = Unbundle By Name(w101) -> ("code"=w113:i32)
              n44 = call "IMAQ ImageToArray"("Image"=w96) -> ("Image Pixels (U16)"=w95:u16[][])  [unwired: 2 in, 5 out]
              n45 = case shown="0, Default" w113 {
                tunnel: w101 -> [w118 w122]
                tunnel: [w118 w121] -> w88
                tunnel: [FALSE TRUE] -> w114
                tunnel: w84 -> [w116 w120]
                tunnel: [w115 w119] -> w97
                frame 0, Default {
                  n46 = Increment(x=w116) -> (x+1=w115:i32)
                }
                frame -1074364414, -1074360293 {
                  n47 = case shown="0" w120 {
                    tunnel: [w124 w130] -> w121
                    tunnel: w122 -> [w126 w130]
                    tunnel: w120 -> [w125 w129]
                    tunnel: [w125 w128] -> w119
                    frame 0 {
                      n48 = Bundle By Name(cluster=w126, "status"=FALSE) -> (w124:errorcluster)
                    }
                    frame 1, Default {
                      n49 = Increment(x=w129) -> (x+1=w128:i32)
                    }
                  }
                }
              }
              "Timeout" <- w114
              n50 = Subtract(x=w82, y=w109) -> (x-y=w110:u32)
              n51 = Not Equal?(x=u32 1, y=w110) -> (x != y?=→"Trigger Overrun":bool)
              n52 = Replace Array Subset(array=w106, new element=w95, index (dim 0)=w84) -> (w105:u16[][][])  [unwired: 2 in]
              n53 = Unbundle By Name(w88) -> ("status"=w108:bool)
              n54 = Greater?(x=4, y=w97) -> (0:w98:bool)
              n55 = Not(x=w108) -> (.not. x?=w107:bool)
              n56 = call "GetStatusInfo.vi"("error in"=w88, "Camera In"=w89) -> ("Status Info"=w83:T8, "error out"=w87:errorcluster, "Camera Out"=w90:T1)  [unwired: 1 in]
              n57 = And(x=w107, y=w98) -> (x .and. y?=w94:bool)
              n58 = Not(x="Interrupt") -> (.not. x?=w91:bool)
              n59 = Insert Into Array(array=w86, new element=w83) -> (w85:T4)  [unwired: 1 in]
              n60 = local write "Camera Error"(w87) -> ()
              n61 = And(x=w94, y=w91) -> (x .and. y?=w93:bool)
              "Frames" <- w84
            }
            "Status Array" <- w44
            n62 = Scale By Power Of 2(n="Bits to shift", x=w61) -> (x*2^n=w60:u16[][][])
            "Images" <- w60
            n63 = call <vilib>:"IMAQdx Unconfigure Acquisition.vi"("error in"=w41, "Session In"=w43) -> ("error out"=w40:errorcluster, "Session Out"=w42:T1)  [unwired: 8 in]
            n64 = call <vilib>:"IMAQdx Close Camera.vi"("error in"=w40, "Session In"=w42) -> ("error out"=w65:errorcluster)  [unwired: 9 out]
          }
          frame #2 {
            # "Transpose for some axes"
            n65 = for {
              tunnel: w132 -> [w134] mode=indexing
              tunnel: [w133] -> w131 mode=indexing
              n66 = local read "Image direction"() -> (w135:enum16{"XY", "XZ"})
              n67 = case shown="\"XY\"" w135 {
                selector: w135 -> [_ w137]
                tunnel: w134 -> [w136 w139]
                tunnel: [w136 w140] -> w133
                frame Default {
                }
                frame "XY" {
                  n68 = case shown="\"XY\"" w137 {
                    tunnel: w139 -> [w141 w143]
                    tunnel: [w141 w142] -> w138
                    frame Default {
                    }
                    frame "XY" {
                      n69 = Transpose 2D Array(2D array=w143) -> (transposed array=w142:u16[][])
                    }
                  }
                  n70 = for {
                    tunnel: w138 -> [w145] mode=indexing
                    tunnel: [w144] -> w140 mode=indexing
                    n71 = Reverse 1D Array(array=w145) -> (reversed array=w144:u16[])
                  }
                }
              }
            }
          }
          frame #3 {
            # "Send to igor a single frame with three images"
            # "For Display only"
            n72 = Array Subset(array=w149, index (dim 0)=1 ("index"), length (dim 0)=3 ("length")) -> (w146:u16[][][])  [unwired: 4 in]
            n73 = Array Size(array=w146) -> (size(s)=w154:i32[])
            n74 = To Single Precision Float(number=w146) -> (single precision float=w155:sgl[][][])
            n75 = case shown="\"Absorption\", Default" "Imaging technique" {
              tunnel: [w167 w173] -> w159
              tunnel: w155 -> [w166 w174]
              frame "Absorption", Default {
                n76 = Index Array(array=w166, index (dim 0)=0 ("Number of buffers")) -> (element=w165:sgl[][])  [unwired: 2 in]
                n77 = Index Array(array=w166, index (dim 0)=1 ("Number of buffers")) -> (element=w164:sgl[][])  [unwired: 2 in]
                n78 = Index Array(array=w166, index (dim 0)=2 ("Number of buffers")) -> (element=w163:sgl[][])  [unwired: 2 in]
                n79 = Subtract(x=w164, y=w163) -> (x-y=w162:sgl[][])
                n80 = Subtract(x=w165, y=w163) -> (x-y=w161:sgl[][])
                n81 = Divide(x=w161, y=w162) -> (x/y=w167:sgl[][])
              }
              frame "Fluorescence" {
                n82 = Index Array(array=w174, index (dim 0)=0 ("Number of buffers")) -> (element=w172:sgl[][])  [unwired: 2 in]
                n83 = Index Array(array=w174, index (dim 0)=1 ("Number of buffers")) -> (element=w171:sgl[][])  [unwired: 2 in]
                n84 = Index Array(array=w174, index (dim 0)=2 ("Number of buffers")) -> ()  [unwired: 2 in, 1 out]
                n85 = Subtract(x=w172, y=w171) -> (x-y=w173:sgl[][])
              }
            }
            "Processed Image" <- w159
            n86 = Index Array(array=w154, index=1 ("Number of buffers")) -> (element=w151:i32)
            n87 = Index Array(array=w154, index=2 ("Number of buffers")) -> (element=w150:i32)
            n88 = Multiply(x=w151, y=3 ("Number of buffers")) -> (x*y=w156:i32)
            n89 = Reshape Array(w146, w156, w150) -> (w158:u16[][])
          }
          frame #4 {
            # "Raw indicates that\nlabview is sending\nthree images"
            n90 = Index String Array(1:"Experiment", 2:string[] ["Experiment=Rubidium_I\n", "Experiment=Rubidium_II\n", "Experiment=RbLi\n\n", "Experiment=RbYb\n", "Experiment=Sr\n"], 3:"") -> (0:w182:string)
            n91 = case shown="True" "Accept parameters from remote system" {
              tunnel: w185 -> [_ w223]
              tunnel: [w199 w215] -> w189
              tunnel: "Experiment" -> [w198 _]
              frame False {
                n92 = case shown="\"Rubidium II\"" w198 {
                  tunnel: [w200 w211] -> w199
                  frame "Rubidium I", Default {
                    # "Build IGOR note string"
                    n93 = Format Into String(format string="I_Race=%e\nI_Pinch=%e\nI_Bias=%e\nt_Expand=%e\nTrap_Min=%e\nDetuning=%e\n", "Racetrack (Amps)", "Pinch Coil (Amps)", "Bias (Amps)", "Expansion time (ms)", "Trap min at 0 (MHz)", "Detuning (Linewidths)") -> (resulting string=w200:string)  [unwired: 2 in, 1 out]
                  }
                  frame "Rubidium II" {
                    # "Build IGOR note string"
                    n94 = local read "Expansion time (ms)"() -> (w209:dbl)
                    n95 = local read "Detuning (Linewidths)"() -> (w208:dbl)
                    n96 = local read "Bias (Amps)"() -> (w210:dbl)
                    n97 = Format Into String(format string="I_Quad=%e\nI_Bias=%e\nt_Expand=%e\nDetuning=%e\n", "Quad [Amps]", w210, w209, w208) -> (resulting string=w211:string)  [unwired: 2 in, 1 out]
                  }
                }
              }
              frame True {
                # "Check for remotly specified paramaters"
                # "Get the remotely created data string"
                # "Search For the remotly specified\nfile number"
                n98 = call "Network_Get_Shared_Variables_v4.vi"("error in (no error)"=w223, "Source of Data"="Source of File Data") -> ("Igor Instruction String"=w222:string[])  [unwired: 1 out]
                n99 = Array To Spreadsheet String(delimiter (Tab)="\n", array=w222, 3:"%s") -> (spreadsheet string=w215:string)
                n100 = Search/Split String(string=w215, search string/char (-)="FileNumber=") -> (match + rest of string=w218:string, offset of match=w217:i32)  [unwired: 2 out]
                n101 = Less Than 0?(x=w217) -> (x < 0?=w216:bool)
                n102 = case shown="False" w216 {
                  tunnel: w218 -> [w228 _]
                  frame False {
                    n103 = Scan From String(format string="FileNumber=%d", input string=w228) -> (output 1=w224:i32)  [unwired: 2 in, 4 out]
                    n104 = local read "File Parameters"() -> (w226:T3)
                    n105 = Bundle By Name(cluster=w226, "Index"=w224) -> (w225:T3)
                    n106 = local write "File Parameters"(w225) -> ()
                  }
                  frame True {
                  }
                }
              }
            }
            n107 = local read "Imaging technique"() -> (w194:enum16{"Absorption", "Fluorescence", "RawImage"})
            n108 = Concatenate Strings(w182, "Camera_ID=Flea3_20S4M\n", "ImageType=Raw\n") -> (w183:string)
            n109 = Index String Array(1:w194, 2:string[] ["DataType=Absorption\n", "DataType=Fluorescence\n", "DataType=RawImage\n"], 3:w183) -> (0:w195:string)
            n110 = Index String Array(1:"Image direction", 2:string[] ["ImageDirection=XY\n", "ImageDirection=XZ\n"], 3:w195) -> (0:w197:string)
            n111 = Format Into String(format string="Magnification=%e\n", initial string=w197, "Magnification") -> (resulting string=w191:string)  [unwired: 1 in, 1 out]
            n112 = Concatenate Strings(w191, w189) -> (→"Image note":string)
          }
          frame #5 {
            # "Save the file as an igor binary"
            n113 = call "MakeFileName_NIST.vi"("File Parameters"="File Parameters", "Save permanent file?"="Save file to archive?") -> ("New file parameters."=w235:T3, "Path to File"=w237:path, "path"=w236:path)
            n114 = local write "File Parameters"(w235) -> ()
            n115 = call "RecursiveMakeDirectory.vi"("Directory to create"=w236) -> ("error out"=w239:errorcluster)  [unwired: 1 in, 1 out]
            n116 = local read "Image note"() -> (w232:string)
            n117 = Delete(path (use dialog)=w237, error in=w239) -> (deleted path=w230:path)  [unwired: 5 out]
            n118 = call "2D INT16 to Igor Binary File.vi"("Wave Data (I16)"=w233, "Wave Note (\"\")"=w232, "WaveName"="Igor Wave Name", "Path (default: dialog)"=w230) -> ("Path chosen"=w229:path)
          }
          frame #6 {
            # "Be sure the file is written"
            n119 = Wait (ms)(milliseconds to wait=u32 1000) -> ()  [unwired: 1 out]
          }
          frame #7 {
            n120 = case shown="True" "Send data to Igor?" {
              tunnel: w243 -> [_ w252]
              tunnel: ["" w251] -> w242
              frame False {
              }
              frame True {
                # "Tell Igor what file to open"
                n121 = Path To String(path=w252) -> (string=w249:string)
                n122 = call <vilib>:"DDE Open Conversation.vi"("topic"="Igor", "service"="Igor") -> ("error out"=w256:errorcluster, "conversation refnum"=w254:u32)  [unwired: 1 in, 5 out]
                n123 = Search and Replace String(replace all?=TRUE, input string=w249, search string="\\", replace string="\\\\") -> (result string=w250:string)  [unwired: 1 in, 6 out]
                n124 = Format Into String(format string="AutoRunV3(\"Sr88_opt\",\"%s\") ", w250) -> (resulting string=w251:string)  [unwired: 2 in, 1 out]
                n125 = call <vilib>:"DDE Execute.vi"("error in (no error)"=w256, "command"=w251, "conversation refnum in"=w254) -> ("error out"=w255:errorcluster, "conversation refnum out"=w253:u32)  [unwired: 5 out]
                n126 = call <vilib>:"DDE Close Conversation.vi"("error in (no error)"=w255, "conversation refnum"=w253) -> ("error out"=→"DDE Error":errorcluster)  [unwired: 7 out]
              }
            }
            "Command to Igor" <- w242
          }
        }
        "Loop" <- w22
      }
    }
    frame #2 {
      n127 = local write "Status"("Done.") -> ()
      "Camera Error" <- w261
    }
    frame #3 {
      n128 = Stop() -> ()  [unwired: 1 out]
    }
  }
  n129 = while {
    stop <- TRUE continue-if-true
    n130 = event shown="[0] \"Raw image to view\", \"Images\", \"Update Graphics\": Value Change;  Timeout" {
      selector: _ -> [_ _]
      dyn-events: _ -> [_ _]
      timeout: 1000 -> [_ _]
      event "Raw image to view", "Images", "Update Graphics": Value Change; Timeout {
        n131 = event-data() -> ()  [unwired: 4 out]
        n132 = case shown="True" "Update Graphics" {
          frame False {
          }
          frame True {
            n133 = local read "Images"() -> (w277:u16[][][])
            n134 = Index Array(array=w277, index (dim 0)="Raw image to view") -> (element=w275:u16[][])  [unwired: 2 in]
            "Raw Image" <- w275
            n135 = Array Size(array=w275) -> (size(s)=w274:i32[])
            n136 = Multiply Array Elements(1:w274) -> (0:w273:i32)
            n137 = Reshape Array(w275, w273) -> (w271:u16[])
            n138 = call <vilib>:"Histogram.vi"("intervals"=64, "X"=w271) -> ("Histogram Graph"=w270:T9)  [unwired: 9 out]
            n139 = Unbundle By Name(w270) -> ("X Values"=w268:dbl[], "Histogram: h(x)"=w269:i32[])
            n140 = Logarithm Base 10(1:w269) -> (0:w267:dbl[])
            n141 = Bundle("X Values"=w268, w267) -> (→"Histogram":cluster{"X Values":dbl[], dbl[]})  [unwired: 1 out]
          }
        }
      }
      event Value Change {
        n142 = event-data() -> ("NewVal"=w278:T3)  [unwired: 6 out]
        n143 = Unbundle By Name(w278) -> ("Index"=w279:u32)
        n144 = global write "FileInfo_Global.vi" "File Index"(w279) -> ()
      }
    }
  }
